vi "Dresden R2R Sputter 03.02.2018 IY24.vi"() -> ()   [LabVIEW 2009] (continued)
        n5019 = case shown="True" w7481 {
          frame #0 {
          }
          frame #1 {
            "ch1_trns_gv_bp2_timer_top" <- TRUE
          }
        }
        n5020 = case shown="True" w7485 {
          frame #0 {
          }
          frame #1 {
            "Gv_timer_top_ch1_2" <- TRUE
          }
        }
        n5021 = case shown="True" w7483 {
          frame #0 {
          }
          frame #1 {
            "ch1_cc_timer_top" <- TRUE
          }
        }
        n5022 = case shown="True" w7482 {
          frame #0 {
          }
          frame #1 {
            "ch1_bg_bv_timer_top" <- TRUE
          }
        }
        n5023 = case shown="True" w7438 {
          frame #0 {
          }
          frame #1 {
            "ch1_sov_Ar_timer_top" <- TRUE
          }
        }
        n5024 = local read "ch1_trns_gv_bp2_timer_top"() -> (w7460:bool)
        n5025 = local read "ch1_bg_bv_timer_top"() -> (w7458:bool)
        n5026 = local read "ch1_sov_Ar_timer_top"() -> (w7440:bool)
        n5027 = local read "Gv_timer_top_ch1_2"() -> (w7461:bool)
        n5028 = Build Array(TRUE, w7484, w7474, w7473, w7472, w7471, w7470, w7451, w7439, w7443, w7417, w7416, w7415) -> (w7524:bool[])
        n5029 = local read "ch1_cc_timer_top"() -> (w7459:bool)
        n5030 = Boolean Array To Number(Boolean array=w7524) -> (number=w7532:u32)
        n5031 = feedback #140() -> (w7468:bool)  [unwired: 1 in]
        n5032 = feedback #141() -> (w7467:bool)  [unwired: 1 in]
        n5033 = feedback #142() -> (w7463:bool)  [unwired: 1 in]
        n5034 = feedback #143() -> (w7441:bool)  [unwired: 1 in]
        n5035 = feedback #144() -> (w7464:bool)  [unwired: 1 in]
        n5036 = Mantissa & Exponent(0:w7532) -> (2:w7528:dbl)  [unwired: 1 out]
        n5037 = case shown="True" w7461 {
          tunnel: [TRUE FALSE] -> w7469
          tunnel: w7468 -> [_ w7585]
          frame #0 {
          }
          frame #1 {
            n5038 = call "Elapsed Time80"("Reset"=w7585) -> ("Elapsed Time (s)"=w7582:dbl)  [unwired: 11 in, 7 out]
            n5039 = Greater?(x=w7582, y=3.0) -> (0:w7583:bool)
            n5040 = In Range and Coerce(upper limit=3.0, x=w7582, lower limit=0.0) -> (In Range?=w7579:bool)  [unwired: 1 out]
            n5041 = Not(x=w7583) -> (.not. x?=w7578:bool)
            n5042 = property on="Gv_timer_top_ch1_2_gui" class="TabCtl (strict)"("Visible"=w7579) -> ()  [unwired: 2 in, 2 out]
            n5043 = local write "Gv_timer_top_ch1_2"(w7578) -> ()
          }
        }
        n5044 = case shown="True" w7460 {
          tunnel: [TRUE FALSE] -> w7466
          tunnel: w7467 -> [_ w7575]
          frame #0 {
          }
          frame #1 {
            n5045 = call "Elapsed Time81"("Reset"=w7575) -> ("Elapsed Time (s)"=w7572:dbl)  [unwired: 11 in, 7 out]
            n5046 = Greater?(x=w7572, y=3.0) -> (0:w7573:bool)
            n5047 = In Range and Coerce(upper limit=3.0, x=w7572, lower limit=0.0) -> (In Range?=w7569:bool)  [unwired: 1 out]
            n5048 = Not(x=w7573) -> (.not. x?=w7568:bool)
            n5049 = local write "ch1_trns_gv_bp2_timer_top"(w7568) -> ()
            n5050 = property on="Ch1_trns_gb_bp2_timer_top_gui" class="TabCtl (strict)"("Visible"=w7569) -> ()  [unwired: 2 in, 2 out]
          }
        }
        n5051 = case shown="True" w7458 {
          tunnel: [TRUE FALSE] -> w7462
          tunnel: w7463 -> [_ w7555]
          frame #0 {
          }
          frame #1 {
            n5052 = call "Elapsed Time83"("Reset"=w7555) -> ("Elapsed Time (s)"=w7552:dbl)  [unwired: 11 in, 7 out]
            n5053 = Greater?(x=w7552, y=3.0) -> (0:w7553:bool)
            n5054 = In Range and Coerce(upper limit=3.0, x=w7552, lower limit=0.0) -> (In Range?=w7548:bool)  [unwired: 1 out]
            n5055 = Not(x=w7553) -> (.not. x?=w7549:bool)
            n5056 = property on="Ch1_bg_bv_timer_top_gui" class="TabCtl (strict)"("Visible"=w7548) -> ()  [unwired: 2 in, 2 out]
            n5057 = local write "ch1_bg_bv_timer_top"(w7549) -> ()
          }
        }
        n5058 = case shown="True" w7440 {
          tunnel: [TRUE FALSE] -> w7442
          tunnel: w7441 -> [_ w7544]
          frame #0 {
          }
          frame #1 {
            n5059 = call "Elapsed Time119"("Reset"=w7544) -> ("Elapsed Time (s)"=w7541:dbl)  [unwired: 11 in, 7 out]
            n5060 = Greater?(x=w7541, y=3.0) -> (0:w7542:bool)
            n5061 = In Range and Coerce(upper limit=3.0, x=w7541, lower limit=0.0) -> (In Range?=w7537:bool)  [unwired: 1 out]
            n5062 = Not(x=w7542) -> (.not. x?=w7538:bool)
            n5063 = property on="Ch1_sov_Ar_timer_top_gui" class="TabCtl (strict)"("Visible"=w7537) -> ()  [unwired: 2 in, 2 out]
            n5064 = local write "ch1_sov_Ar_timer_top"(w7538) -> ()
          }
        }
        n5065 = case shown="True" w7459 {
          tunnel: [TRUE FALSE] -> w7465
          tunnel: w7464 -> [_ w7565]
          frame #0 {
          }
          frame #1 {
            n5066 = call "Elapsed Time82"("Reset"=w7565) -> ("Elapsed Time (s)"=w7562:dbl)  [unwired: 11 in, 7 out]
            n5067 = Greater?(x=w7562, y=3.0) -> (0:w7563:bool)
            n5068 = In Range and Coerce(upper limit=3.0, x=w7562, lower limit=0.0) -> (In Range?=w7559:bool)  [unwired: 1 out]
            n5069 = Not(x=w7563) -> (.not. x?=w7558:bool)
            n5070 = local write "ch1_cc_timer_top"(w7558) -> ()
            n5071 = property on="Ch1_cc_timer_top_gui" class="TabCtl (strict)"("Visible"=w7559) -> ()  [unwired: 2 in, 2 out]
          }
        }
        n5072 = case shown="12" w7528 {
          tunnel: [cluster{"x":i16, "y":i16} {"x"=0, "y"=0} ("origin") cluster{"x":i16, "y":i16} {"x"=75, "y"=463} ("origin") cluster{"x":i16, "y":i16} {"x"=198, "y"=269} ("origin") cluster{"x":i16, "y":i16} {"x"=282, "y"=670} ("origin") cluster{"x":i16, "y":i16} {"x"=420, "y"=648} ("origin") cluster{"x":i16, "y":i16} {"x"=491, "y"=687} ("origin") cluster{"x":i16, "y":i16} {"x"=206, "y"=664} ("origin") cluster{"x":i16, "y":i16} {"x"=383, "y"=718} ("origin") cluster{"x":i16, "y":i16} {"x"=502, "y"=186} ("origin") cluster{"x":i16, "y":i16} {"x"=562, "y"=180} ("origin") cluster{"x":i16, "y":i16} {"x"=250, "y"=166} ("origin") cluster{"x":i16, "y":i16} {"x"=414, "y"=166} ("origin") cluster{"x":i16, "y":i16} {"x"=320, "y"=144} ("origin")] -> w7530
          tunnel: ["" ("text") "GV" ("text") "GV-BP" ("text") "CH-CC" ("text") "BG-BV" ("text") "CH-ATM" ("text") "CH-PG" ("text") "CH-BG" ("text") "SOV-Ar" ("text") "MFC" ("text") "CST-FIX" ("text") "CST-FIX" ("text") "PET-COOL" ("text")] -> w7531
          tunnel: ["" ("DESCRIPTION") "Gate Valve" ("DESCRIPTION") "Gate Valve- By Pass" ("DESCRIPTION") "Chamber-Cold Cathode" ("DESCRIPTION") "Baratron Gauge-Block Valve" ("DESCRIPTION") "Chamber-Atmospheric Switch" ("DESCRIPTION") "Chamber-Pirani Gauge" ("DESCRIPTION") "Chamber-Baratron Gauge" ("DESCRIPTION") "Shut Off Valve-Ar Gas" ("DESCRIPTION") "Mass Flow Control" ("DESCRIPTION") "Casette Fix" ("DESCRIPTION") "Casette Fix" ("DESCRIPTION") "Petfolio Cool " ("DESCRIPTION")] -> w7529
          frame #0 {
          }
          frame #1 {
          }
          frame #2 {
          }
          frame #3 {
          }
          frame #4 {
          }
          frame #5 {
          }
          frame #6 {
          }
          frame #7 {
          }
          frame #8 {
          }
          frame #9 {
          }
          frame #10 {
          }
          frame #11 {
          }
          frame #12 {
          }
        }
        n5073 = local write "DESCRIPTION"(w7529) -> ()
        n5074 = call <vilib>:"Draw Text at Point.vi"("[user-specified font]"=T35 {"Font Name:"="BOLD", "Size"=18, "Strikeout?"=FALSE, "Italic?"=FALSE, "Underline?"=FALSE, "Outline?"=FALSE, "Shadow?"=FALSE, "Bold?"=TRUE} ("[user-specified font] 9"), "desired font(Application)"=T36."User-specified Font", "text"=w7531, "origin"=w7530, "picture"=w7527) -> ("new picture"=w7522:picture)  [unwired: 5 in, 1 out]
      }
    }
    "new picture 7" <- w7254
    n5075 = stacked-sequence {
      tunnel: w7282 -> [w7649 _]
      tunnel: [_ w7738] -> w7269
      tunnel: w7281 -> [w7683 _]
      tunnel: w7280 -> [w7681 _]
      tunnel: w7279 -> [w7676 _]
      tunnel: w7278 -> [w7671 _]
      tunnel: w7277 -> [w7670 _]
      tunnel: w7276 -> [w7661 _]
      tunnel: w7275 -> [w7652 _]
      tunnel: w7274 -> [w7651 _]
      tunnel: w7268 -> [w7635 _]
      tunnel: w7267 -> [w7634 _]
      frame #0 {
        n5076 = Build Array(FALSE ("element"), "chamber1 front piston open drum failed", "chamber1 front piston failed drum open", "chamber1 front piston open") -> (w7687:bool[])
        n5077 = Build Array(FALSE ("element"), "magnetron on ch1") -> (w7666:bool[])
        n5078 = Build Array(FALSE ("element"), "gv front open ch1_2", "gv front failed ch1_2") -> (w7679:bool[])
        n5079 = Build Array(FALSE ("element"), "magnetron water cooled on ch1", "magnetron water cooled failed ch1") -> (w7653:bool[])
        n5080 = Build Array(FALSE ("element"), "Trns_gv_bp2_ch1_fail_front", "Trns_gv_bp2_ch1_on_front") -> (w7640:bool[])
        n5081 = Boolean Array To Number(Boolean array=w7687) -> (number=w7686:u32)
        n5082 = Boolean Array To Number(Boolean array=w7666) -> (number=w7665:u32)
        n5083 = Boolean Array To Number(Boolean array=w7679) -> (number=w7680:u32)
        n5084 = Boolean Array To Number(Boolean array=w7653) -> (number=w7654:u32)
        n5085 = Boolean Array To Number(Boolean array=w7640) -> (number=w7639:u32)
        n5086 = Mantissa & Exponent(0:w7686) -> (2:w7685:dbl)  [unwired: 1 out]
        n5087 = Mantissa & Exponent(0:w7665) -> (2:w7662:dbl)  [unwired: 1 out]
        n5088 = Mantissa & Exponent(0:w7680) -> (2:w7675:dbl)  [unwired: 1 out]
        n5089 = Mantissa & Exponent(0:w7654) -> (2:w7657:dbl)  [unwired: 1 out]
        n5090 = Mantissa & Exponent(0:w7639) -> (2:w7636:dbl)  [unwired: 1 out]
        n5091 = case shown="0, Default" w7685 {
          tunnel: [u32[][] [] ("data (RGB format)") w7700 w7701 w7702] -> w7684
          tunnel: w7683 -> [_ w7700 _ _]
          tunnel: w7681 -> [_ _ w7701 _]
          tunnel: w7671 -> [_ _ _ w7702]
          frame #0 {
          }
          frame #1 {
          }
          frame #2 {
          }
          frame #3 {
          }
        }
        n5092 = case shown="0, Default" w7675 {
          tunnel: [u32[][] [] ("data (RGB format)") w7697 w7698] -> w7677
          tunnel: w7676 -> [_ w7697 _]
          tunnel: w7670 -> [_ _ w7698]
          frame #0 {
          }
          frame #1 {
          }
          frame #2 {
          }
        }
        n5093 = case shown="0, Default" w7662 {
          tunnel: w7661 -> [_ w7695]
          tunnel: [u32[][] [] ("data (RGB format)") w7695] -> w7659
          frame #0 {
          }
          frame #1 {
          }
        }
        n5094 = case shown="0, Default" w7657 {
          tunnel: w7652 -> [_ w7692 _]
          tunnel: [u32[][] [] ("data (RGB format)") w7692 w7693] -> w7658
          tunnel: w7651 -> [_ _ w7693]
          frame #0 {
          }
          frame #1 {
          }
          frame #2 {
          }
        }
        n5095 = case shown="0, Default" w7636 {
          tunnel: w7635 -> [_ w7689 _]
          tunnel: [u32[][] [] ("data (RGB format)") w7689 w7690] -> w7631
          tunnel: w7634 -> [_ _ w7690]
          frame #0 {
          }
          frame #1 {
          }
          frame #2 {
          }
        }
        n5096 = call-poly <vilib>:"Draw Unflattened Pixmap.vi"("top left point(0, 0)"=cluster{"x":i16, "y":i16} {"x"=100, "y"=167}, "data (RGB format)"=w7649) -> ("new picture"=w7647:picture)  [unwired: 7 in]
        n5097 = call-poly <vilib>:"Draw Unflattened Pixmap.vi"("picture"=w7647, "top left point(0, 0)"=cluster{"x":i16, "y":i16} {"x"=187, "y"=296} ("top left point(0, 0) 3"), "data (RGB format)"=w7684) -> ("new picture"=w7678:picture)  [unwired: 6 in]
        n5098 = call-poly <vilib>:"Draw Unflattened Pixmap.vi"("picture"=w7678, "top left point(0, 0)"=cluster{"x":i16, "y":i16} {"x"=98, "y"=311} ("top left point(0, 0) 2"), "data (RGB format)"=w7677) -> ("new picture"=w7660:picture)  [unwired: 6 in]
        n5099 = call-poly <vilib>:"Draw Unflattened Pixmap.vi"("picture"=w7660, "top left point(0, 0)"=cluster{"x":i16, "y":i16} {"x"=296, "y"=587}, "data (RGB format)"=w7659) -> ("new picture"=w7648:picture)  [unwired: 6 in]
        n5100 = call-poly <vilib>:"Draw Unflattened Pixmap.vi"("picture"=w7648, "top left point(0, 0)"=cluster{"x":i16, "y":i16} {"x"=316, "y"=647}, "data (RGB format)"=w7658) -> ("new picture"=w7632:picture)  [unwired: 6 in]
        n5101 = call-poly <vilib>:"Draw Unflattened Pixmap.vi"("picture"=w7632, "top left point(0, 0)"=cluster{"x":i16, "y":i16} {"x"=182, "y"=249}, "data (RGB format)"=w7631) -> ("new picture"=w7633:picture)  [unwired: 6 in]
      }
      frame #1 {
        # "PET COOL"
        # "CST-FIX"
        # "CST-FIX"
        n5102 = property on="new picture 8" class="Pict"() -> ("Mouse"=w7737:T37)  [unwired: 2 in, 2 out]
        n5103 = Unbundle(w7737) -> ("Mouse Position"=w7736:cluster{"X":i32, "Y":i32}, "Mouse Modifiers"=w7735:T38)
        "Mouse Position 8" <- w7736
        n5104 = Unbundle(w7736) -> ("X"=w7704:i32, "Y"=w7703:i32)
        n5105 = Unbundle(w7735) -> ("Button Down"=w7734:bool)  [unwired: 3 out]
        n5106 = In Range and Coerce(upper limit=598, x=w7703, lower limit=319) -> (In Range?=w7764:bool)  [unwired: 1 out]
        n5107 = In Range and Coerce(upper limit=146, x=w7704, lower limit=106) -> (In Range?=w7765:bool)  [unwired: 1 out]
        n5108 = In Range and Coerce(upper limit=275, x=w7703, lower limit=204) -> (In Range?=w7763:bool)  [unwired: 1 out]
        n5109 = In Range and Coerce(upper limit=225, x=w7704, lower limit=192) -> (In Range?=w7762:bool)  [unwired: 1 out]
        n5110 = In Range and Coerce(upper limit=331, x=w7703, lower limit=169) -> (In Range?=w7713:bool)  [unwired: 1 out]
        n5111 = In Range and Coerce(upper limit=382, x=w7704, lower limit=342) -> (In Range?=w7712:bool)  [unwired: 1 out]
        n5112 = In Range and Coerce(upper limit=679, x=w7703, lower limit=639) -> (In Range?=w7752:bool)  [unwired: 1 out]
        n5113 = In Range and Coerce(upper limit=324, x=w7703, lower limit=201) -> (In Range?=w7714:bool)  [unwired: 1 out]
        n5114 = In Range and Coerce(upper limit=425, x=w7704, lower limit=303) -> (In Range?=w7753:bool)  [unwired: 1 out]
        n5115 = In Range and Coerce(upper limit=471, x=w7704, lower limit=446) -> (In Range?=w7715:bool)  [unwired: 1 out]
        n5116 = In Range and Coerce(upper limit=324, x=w7703, lower limit=201) -> (In Range?=w7725:bool)  [unwired: 1 out]
        n5117 = In Range and Coerce(upper limit=275, x=w7704, lower limit=247) -> (In Range?=w7724:bool)  [unwired: 1 out]
        n5118 = And(x=w7765, y=w7764) -> (x .and. y?=w7745:bool)
        n5119 = And(x=w7762, y=w7763) -> (x .and. y?=w7733:bool)
        n5120 = And(x=w7712, y=w7713) -> (x .and. y?=w7705:bool)
        n5121 = And(x=w7753, y=w7752) -> (x .and. y?=w7732:bool)
        n5122 = And(x=w7715, y=w7714) -> (x .and. y?=w7706:bool)
        n5123 = And(x=w7724, y=w7725) -> (x .and. y?=w7707:bool)
        n5124 = And(x=w7734, y=w7745) -> (x .and. y?=w7747:bool)
        n5125 = And(x=w7734, y=w7733) -> (x .and. y?=w7744:bool)
        n5126 = case shown="True" w7747 {
          frame #0 {
          }
          frame #1 {
            "Gv_timer_front_ch1_2" <- TRUE ("Gv_timer_front_ch2_3")
          }
        }
        n5127 = case shown="True" w7744 {
          frame #0 {
          }
          frame #1 {
            "ch1_trns_gv_bp2_timer_front" <- TRUE ("ch2_bv_L_timerl_front")
          }
        }
        n5128 = Build Array(TRUE, w7745, w7733, w7732, w7707, w7706, w7705) -> (w7748:bool[])
        n5129 = local read "ch1_trns_gv_bp2_timer_front"() -> (w7726:bool)
        n5130 = local read "Gv_timer_front_ch1_2"() -> (w7727:bool)
        n5131 = Boolean Array To Number(Boolean array=w7748) -> (number=w7751:u32)
        n5132 = Mantissa & Exponent(0:w7751) -> (2:w7740:dbl)  [unwired: 1 out]
        n5133 = feedback #145() -> (w7728:bool)  [unwired: 1 in]
        n5134 = feedback #146() -> (w7730:bool)  [unwired: 1 in]
        n5135 = case shown="True" w7726 {
          tunnel: [TRUE FALSE] -> w7729
          tunnel: w7728 -> [_ w7778]
          frame #0 {
          }
          frame #1 {
            n5136 = call "Elapsed Time79"("Reset"=w7778) -> ("Elapsed Time (s)"=w7775:dbl)  [unwired: 11 in, 7 out]
            n5137 = Greater?(x=w7775, y=3.0) -> (0:w7776:bool)
            n5138 = In Range and Coerce(upper limit=3.0, x=w7775, lower limit=0.0) -> (In Range?=w7772:bool)  [unwired: 1 out]
            n5139 = Not(x=w7776) -> (.not. x?=w7771:bool)
            n5140 = local write "ch1_trns_gv_bp2_timer_front"(w7771) -> ()
            n5141 = property on="Ch1_trns_gv_bp2_timer_front_gui" class="TabCtl (strict)"("Visible"=w7772) -> ()  [unwired: 2 in, 2 out]
          }
        }
        n5142 = case shown="True" w7727 {
          tunnel: [TRUE FALSE] -> w7731
          tunnel: w7730 -> [_ w7788]
          frame #0 {
          }
          frame #1 {
            n5143 = call "Elapsed Time78"("Reset"=w7788) -> ("Elapsed Time (s)"=w7785:dbl)  [unwired: 11 in, 7 out]
            n5144 = Greater?(x=w7785, y=3.0) -> (0:w7786:bool)
            n5145 = In Range and Coerce(upper limit=3.0, x=w7785, lower limit=0.0) -> (In Range?=w7782:bool)  [unwired: 1 out]
            n5146 = Not(x=w7786) -> (.not. x?=w7781:bool)
            n5147 = local write "Gv_timer_front_ch1_2"(w7781) -> ()
            n5148 = property on="Gv_timer_front_ch1_2_gui" class="TabCtl (strict)"("Visible"=w7782) -> ()  [unwired: 2 in, 2 out]
          }
        }
        n5149 = case shown="6" w7740 {
          tunnel: [cluster{"x":i16, "y":i16} {"x"=0, "y"=0} ("origin") cluster{"x":i16, "y":i16} {"x"=71, "y"=502} ("origin") cluster{"x":i16, "y":i16} {"x"=186, "y"=231} ("origin") cluster{"x":i16, "y":i16} {"x"=353, "y"=707} ("origin") cluster{"x":i16, "y":i16} {"x"=231, "y"=185} ("origin") cluster{"x":i16, "y":i16} {"x"=440, "y"=185} ("origin") cluster{"x":i16, "y":i16} {"x"=327, "y"=149} ("origin")] -> w7742
          tunnel: ["" ("text") "GV" ("text") "GV-BP" ("text") "MG" ("text") "CST-FIX" ("text") "CST-FIX" ("text") "PET-COOL" ("text")] -> w7743
          tunnel: ["" ("DESCRIPTION") "Gate Valve" ("DESCRIPTION") "Gate Valve- By Pass" ("DESCRIPTION") "MAGNETRON" ("DESCRIPTION") "Casette Fix" ("DESCRIPTION") "Casette Fix" ("DESCRIPTION") "Petfolio Cool " ("DESCRIPTION")] -> w7741
          frame #0 {
          }
          frame #1 {
          }
          frame #2 {
          }
          frame #3 {
          }
          frame #4 {
          }
          frame #5 {
          }
          frame #6 {
          }
        }
        n5150 = local write "DESCRIPTION"(w7741) -> ()
        n5151 = call <vilib>:"Draw Text at Point.vi"("[user-specified font]"=T35 {"Font Name:"="BOLD", "Size"=18, "Strikeout?"=FALSE, "Italic?"=FALSE, "Underline?"=FALSE, "Outline?"=FALSE, "Shadow?"=FALSE, "Bold?"=TRUE} ("[user-specified font] 8"), "desired font(Application)"=T36."User-specified Font", "text"=w7743, "origin"=w7742, "picture"=w7739) -> ("new picture"=w7738:picture)  [unwired: 5 in, 1 out]
      }
    }
    "new picture 8" <- w7269
  }
  n5152 = while {
    tunnel: w557 -> [w7853]
    tunnel: w556 -> [w7852]
    tunnel: w555 -> [w7851]
    tunnel: w554 -> [w7850]
    tunnel: w553 -> [w7849]
    tunnel: w552 -> [w7848]
    tunnel: w551 -> [w7847]
    tunnel: w550 -> [w7846]
    tunnel: w549 -> [w7845]
    tunnel: w548 -> [w7844]
    tunnel: w547 -> [w7843]
    tunnel: w546 -> [w7842]
    tunnel: w545 -> [w7841]
    tunnel: w544 -> [w7840]
    tunnel: w225 -> [w7838]
    tunnel: w224 -> [w7837]
    tunnel: w175 -> [w7836]
    tunnel: w174 -> [w7835]
    tunnel: w173 -> [w7834]
    tunnel: w172 -> [w7833]
    tunnel: w171 -> [w7832]
    tunnel: w170 -> [w7831]
    tunnel: w169 -> [w7830]
    tunnel: w168 -> [w7829]
    tunnel: w167 -> [w7828]
    tunnel: w166 -> [w7827]
    tunnel: w165 -> [w7826]
    tunnel: w164 -> [w7825]
    tunnel: w163 -> [w7824]
    tunnel: w162 -> [w7823]
    tunnel: w161 -> [w7822]
    tunnel: w160 -> [w7821]
    tunnel: w126 -> [w7820]
    tunnel: w125 -> [w7819]
    tunnel: w111 -> [w7818]
    tunnel: w110 -> [w7817]
    tunnel: w109 -> [w7816]
    tunnel: w108 -> [w7815]
    stop <- FALSE stop-if-true
    n5153 = stacked-sequence {
      tunnel: w7853 -> [w8340 _]
      tunnel: w7852 -> [w8339 _]
      tunnel: w7851 -> [w8338 _]
      tunnel: w7850 -> [w8337 _]
      tunnel: w7849 -> [w8335 _]
      tunnel: w7848 -> [w8336 _]
      tunnel: w7847 -> [w8334 _]
      tunnel: w7846 -> [w8333 _]
      tunnel: w7845 -> [w8332 _]
      tunnel: [_ w8433] -> w7839
      tunnel: w7838 -> [w8311 _]
      tunnel: w7837 -> [w8310 _]
      tunnel: w7818 -> [w8285 _]
      tunnel: w7817 -> [w8284 _]
      tunnel: w7816 -> [w8283 _]
      tunnel: w7815 -> [w8282 _]
      frame #0 {
        n5154 = Build Array(FALSE ("element"), "ch2_trns_gv_bp2_on_front", "ch2_trns_gv_bp2_fail_front") -> (w8296:bool[])
        n5155 = Build Array(FALSE ("element"), "magnetron on_ch3") -> (w8354:bool[])
        n5156 = Build Array(FALSE ("element"), "chamber2 front piston failed drum open", "chamber2 front piston open drum failed", "chamber2front piston open") -> (w8344:bool[])
        n5157 = Build Array(FALSE ("element"), "gv front open_ch2_3", "gv front failed_ch2_3") -> (w8357:bool[])
        n5158 = Build Array(FALSE ("element"), "ch2_trns_gv_bp_fail_front", "ch2_trns_gv_bp_on_front") -> (w8291:bool[])
        n5159 = Build Array(FALSE ("element"), "magnetron water cooled on_ch2", "magnetron water cooled failed_ch2") -> (w8346:bool[])
        n5160 = Build Array(FALSE ("element"), "gv front failed_ch2_1", "gv front open_ch2_1") -> (w8312:bool[])
        n5161 = Boolean Array To Number(Boolean array=w8296) -> (number=w8297:u32)
        n5162 = Boolean Array To Number(Boolean array=w8354) -> (number=w8353:u32)
        n5163 = Boolean Array To Number(Boolean array=w8344) -> (number=w8343:u32)
        n5164 = Boolean Array To Number(Boolean array=w8357) -> (number=w8358:u32)
        n5165 = Boolean Array To Number(Boolean array=w8291) -> (number=w8302:u32)
        n5166 = Boolean Array To Number(Boolean array=w8346) -> (number=w8347:u32)
        n5167 = Boolean Array To Number(Boolean array=w8312) -> (number=w8313:u32)
        n5168 = Mantissa & Exponent(0:w8297) -> (2:w8298:dbl)  [unwired: 1 out]
        n5169 = Mantissa & Exponent(0:w8302) -> (2:w8301:dbl)  [unwired: 1 out]
        n5170 = Mantissa & Exponent(0:w8353) -> (2:w8352:dbl)  [unwired: 1 out]
        n5171 = Mantissa & Exponent(0:w8343) -> (2:w8342:dbl)  [unwired: 1 out]
        n5172 = Mantissa & Exponent(0:w8358) -> (2:w8355:dbl)  [unwired: 1 out]
        n5173 = Mantissa & Exponent(0:w8313) -> (2:w8314:dbl)  [unwired: 1 out]
        n5174 = Mantissa & Exponent(0:w8347) -> (2:w8348:dbl)  [unwired: 1 out]
        n5175 = case shown="1" w8301 {
          tunnel: [u32[][] [] ("data (RGB format)") w8364 w8365] -> w8300
          tunnel: w8285 -> [_ w8364 _]
          tunnel: w8284 -> [_ _ w8365]
          frame #0 {
          }
          frame #1 {
          }
          frame #2 {
          }
        }
        n5176 = case shown="2" w8298 {
          tunnel: [u32[][] [] ("data (RGB format)") w8361 w8362] -> w8299
          tunnel: w8283 -> [_ w8361 _]
          tunnel: w8282 -> [_ _ w8362]
          frame #0 {
          }
          frame #1 {
          }
          frame #2 {
          }
        }
        n5177 = case shown="1" w8342 {
          tunnel: [u32[][] [] ("data (RGB format)") w8378 w8379 w8380] -> w8341
          tunnel: w8339 -> [_ w8378 _ _]
          tunnel: w8338 -> [_ _ w8379 _]
          tunnel: w8337 -> [_ _ _ w8380]
          frame #0 {
          }
          frame #1 {
          }
          frame #2 {
          }
          frame #3 {
          }
        }
        n5178 = case shown="0, Default" w8314 {
          tunnel: w8311 -> [_ w8367 _]
          tunnel: [u32[][] [] ("data (RGB format)") w8367 w8368] -> w8318
          tunnel: w8310 -> [_ _ w8368]
          frame #0 {
          }
          frame #1 {
          }
          frame #2 {
          }
        }
        n5179 = case shown="1" w8355 {
          tunnel: [u32[][] [] ("data (RGB format)") w8375 w8376] -> w8356
          tunnel: w8336 -> [_ _ w8376]
          tunnel: w8335 -> [_ w8375 _]
          frame #0 {
          }
          frame #1 {
          }
          frame #2 {
          }
        }
        n5180 = case shown="1" w8352 {
          tunnel: [u32[][] [] ("data (RGB format)") w8373] -> w8350
          tunnel: w8334 -> [_ w8373]
          frame #0 {
          }
          frame #1 {
          }
        }
        n5181 = case shown="0, Default" w8348 {
          tunnel: w8333 -> [_ w8370 _]
          tunnel: [u32[][] [] ("data (RGB format)") w8370 w8371] -> w8349
          tunnel: w8332 -> [_ _ w8371]
          frame #0 {
          }
          frame #1 {
          }
          frame #2 {
          }
        }
        n5182 = call-poly <vilib>:"Draw Unflattened Pixmap.vi"("top left point(0, 0)"=cluster{"x":i16, "y":i16} {"x"=93, "y"=169}, "data (RGB format)"=w8340) -> ("new picture"=w8331:picture)  [unwired: 7 in]
        n5183 = call-poly <vilib>:"Draw Unflattened Pixmap.vi"("picture"=w8331, "top left point(0, 0)"=cluster{"x":i16, "y":i16} {"x"=182, "y"=297}, "data (RGB format)"=w8341) -> ("new picture"=w8359:picture)  [unwired: 6 in]
        n5184 = call-poly <vilib>:"Draw Unflattened Pixmap.vi"("picture"=w8359, "top left point(0, 0)"=cluster{"x":i16, "y":i16} {"x"=564, "y"=310}, "data (RGB format)"=w8356) -> ("new picture"=w8351:picture)  [unwired: 6 in]
        n5185 = call-poly <vilib>:"Draw Unflattened Pixmap.vi"("picture"=w8351, "top left point(0, 0)"=cluster{"x":i16, "y":i16} {"x"=282, "y"=593}, "data (RGB format)"=w8350) -> ("new picture"=w8345:picture)  [unwired: 6 in]
        n5186 = call-poly <vilib>:"Draw Unflattened Pixmap.vi"("picture"=w8345, "top left point(0, 0)"=cluster{"x":i16, "y":i16} {"x"=304, "y"=649}, "data (RGB format)"=w8349) -> ("new picture"=w8309:picture)  [unwired: 6 in]
        n5187 = call-poly <vilib>:"Draw Unflattened Pixmap.vi"("picture"=w8309, "top left point(0, 0)"=cluster{"x":i16, "y":i16} {"x"=92, "y"=313}, "data (RGB format)"=w8318) -> ("new picture"=w8286:picture)  [unwired: 6 in]
        n5188 = call-poly <vilib>:"Draw Unflattened Pixmap.vi"("picture"=w8286, "top left point(0, 0)"=cluster{"x":i16, "y":i16} {"x"=175, "y"=251}, "data (RGB format)"=w8300) -> ("new picture"=w8287:picture)  [unwired: 6 in]
        n5189 = call-poly <vilib>:"Draw Unflattened Pixmap.vi"("picture"=w8287, "top left point(0, 0)"=cluster{"x":i16, "y":i16} {"x"=488, "y"=250} ("top left point(0, 0) 2"), "data (RGB format)"=w8299) -> ("new picture"=w8288:picture)  [unwired: 6 in]
      }
      frame #1 {
        # "PET COOL"
        # "CST FIX"
        # "CST FIX"
        n5190 = property on="new picture 5" class="Pict"() -> ("Mouse"=w8468:T37)  [unwired: 2 in, 2 out]
        n5191 = Unbundle(w8468) -> ("Mouse Position"=w8467:cluster{"X":i32, "Y":i32}, "Mouse Modifiers"=w8469:T38)
        "Mouse Position 6" <- w8467
        n5192 = Unbundle(w8469) -> ("Button Down"=w8436:bool)  [unwired: 3 out]
        n5193 = Unbundle(w8467) -> ("X"=w8382:i32, "Y"=w8381:i32)
        n5194 = In Range and Coerce(upper limit=333, x=w8381, lower limit=171) -> (In Range?=w8391:bool)  [unwired: 1 out]
        n5195 = In Range and Coerce(upper limit=382, x=w8382, lower limit=327) -> (In Range?=w8390:bool)  [unwired: 1 out]
        n5196 = In Range and Coerce(upper limit=605, x=w8381, lower limit=324) -> (In Range?=w8460:bool)  [unwired: 1 out]
        n5197 = In Range and Coerce(upper limit=140, x=w8382, lower limit=98) -> (In Range?=w8459:bool)  [unwired: 1 out]
        n5198 = In Range and Coerce(upper limit=600, x=w8381, lower limit=324) -> (In Range?=w8461:bool)  [unwired: 1 out]
        n5199 = In Range and Coerce(upper limit=325, x=w8381, lower limit=203) -> (In Range?=w8392:bool)  [unwired: 1 out]
        n5200 = In Range and Coerce(upper limit=610, x=w8382, lower limit=570) -> (In Range?=w8462:bool)  [unwired: 1 out]
        n5201 = In Range and Coerce(upper limit=474, x=w8382, lower limit=435) -> (In Range?=w8393:bool)  [unwired: 1 out]
        n5202 = In Range and Coerce(upper limit=277, x=w8381, lower limit=252) -> (In Range?=w8450:bool)  [unwired: 1 out]
        n5203 = In Range and Coerce(upper limit=527, x=w8382, lower limit=490) -> (In Range?=w8451:bool)  [unwired: 1 out]
        n5204 = In Range and Coerce(upper limit=325, x=w8381, lower limit=203) -> (In Range?=w8403:bool)  [unwired: 1 out]
        n5205 = In Range and Coerce(upper limit=275, x=w8382, lower limit=235) -> (In Range?=w8402:bool)  [unwired: 1 out]
        n5206 = In Range and Coerce(upper limit=281, x=w8381, lower limit=256) -> (In Range?=w8449:bool)  [unwired: 1 out]
        n5207 = In Range and Coerce(upper limit=210, x=w8382, lower limit=185) -> (In Range?=w8448:bool)  [unwired: 1 out]
        n5208 = In Range and Coerce(upper limit=685, x=w8381, lower limit=641) -> (In Range?=w8438:bool)  [unwired: 1 out]
        n5209 = In Range and Coerce(upper limit=418, x=w8382, lower limit=283) -> (In Range?=w8439:bool)  [unwired: 1 out]
        n5210 = And(x=w8390, y=w8391) -> (x .and. y?=w8383:bool)
        n5211 = And(x=w8459, y=w8460) -> (x .and. y?=w8423:bool)
        n5212 = And(x=w8462, y=w8461) -> (x .and. y?=w8427:bool)
        n5213 = And(x=w8393, y=w8392) -> (x .and. y?=w8384:bool)
        n5214 = And(x=w8451, y=w8450) -> (x .and. y?=w8422:bool)
        n5215 = And(x=w8402, y=w8403) -> (x .and. y?=w8385:bool)
        n5216 = And(x=w8448, y=w8449) -> (x .and. y?=w8421:bool)
        n5217 = And(x=w8439, y=w8438) -> (x .and. y?=w8420:bool)
        n5218 = And(x=w8436, y=w8427) -> (x .and. y?=w8429:bool)
        n5219 = And(x=w8436, y=w8423) -> (x .and. y?=w8426:bool)
        n5220 = And(x=w8436, y=w8422) -> (x .and. y?=w8425:bool)
        n5221 = And(x=w8436, y=w8421) -> (x .and. y?=w8424:bool)
        n5222 = case shown="True" w8429 {
          frame #0 {
          }
          frame #1 {
            "Gv_timer_front_ch2_1" <- TRUE ("Gv_timer_front_ch2_3")
          }
        }
        n5223 = case shown="True" w8426 {
          frame #0 {
          }
          frame #1 {
            "Gv_timer_front_ch2_3" <- TRUE ("Gv_timer_front_ch2_1")
          }
        }
        n5224 = case shown="True" w8425 {
          frame #0 {
          }
          frame #1 {
            "ch2_trns_gv_bp_timer_front" <- TRUE ("ch2_bv_R_timer_front")
          }
        }
        n5225 = case shown="True" w8424 {
          frame #0 {
          }
          frame #1 {
            "ch2_trns_gv_bp2_timer_front" <- TRUE ("ch2_bv_L_timerl_front")
          }
        }
        n5226 = Build Array(TRUE, w8427, w8423, w8422, w8421, w8420, w8385, w8384, w8383) -> (w8430:bool[])
        n5227 = local read "ch2_trns_gv_bp_timer_front"() -> (w8405:bool)
        n5228 = local read "Gv_timer_front_ch2_3"() -> (w8406:bool)
        n5229 = local read "ch2_trns_gv_bp2_timer_front"() -> (w8404:bool)
        n5230 = local read "Gv_timer_front_ch2_1"() -> (w8407:bool)
        n5231 = Boolean Array To Number(Boolean array=w8430) -> (number=w8435:u32)
        n5232 = Mantissa & Exponent(0:w8435) -> (2:w8416:dbl)  [unwired: 1 out]
        n5233 = feedback #147() -> (w8414:bool)  [unwired: 1 in]
        n5234 = feedback #148() -> (w8413:bool)  [unwired: 1 in]
        n5235 = feedback #149() -> (w8410:bool)  [unwired: 1 in]
        n5236 = feedback #150() -> (w8409:bool)  [unwired: 1 in]
        n5237 = case shown="True" w8407 {
          tunnel: [TRUE FALSE] -> w8415
          tunnel: w8414 -> [_ w8508]
          frame #0 {
          }
          frame #1 {
            n5238 = call "Elapsed Time67"("Reset"=w8508) -> ("Elapsed Time (s)"=w8505:dbl)  [unwired: 11 in, 7 out]
            n5239 = Greater?(x=w8505, y=3.0) -> (0:w8506:bool)
            n5240 = In Range and Coerce(upper limit=3.0, x=w8505, lower limit=0.0) -> (In Range?=w8501:bool)  [unwired: 1 out]
            n5241 = Not(x=w8506) -> (.not. x?=w8502:bool)
            n5242 = local write "Gv_timer_front_ch2_1"(w8502) -> ()
            n5243 = property on="Gv_timer_front_ch2_1_gui" class="TabCtl (strict)"("Visible"=w8501) -> ()  [unwired: 2 in, 2 out]
          }
        }
        n5244 = case shown="True" w8406 {
          tunnel: [TRUE FALSE] -> w8412
          tunnel: w8413 -> [_ w8498]
          frame #0 {
          }
          frame #1 {
            n5245 = call "Elapsed Time68"("Reset"=w8498) -> ("Elapsed Time (s)"=w8495:dbl)  [unwired: 11 in, 7 out]
            n5246 = Greater?(x=w8495, y=3.0) -> (0:w8496:bool)
            n5247 = In Range and Coerce(upper limit=3.0, x=w8495, lower limit=0.0) -> (In Range?=w8491:bool)  [unwired: 1 out]
            n5248 = Not(x=w8496) -> (.not. x?=w8492:bool)
            n5249 = local write "Gv_timer_front_ch2_3"(w8492) -> ()
            n5250 = property on="Gv_timer_front_ch2_3_gui" class="TabCtl (strict)"("Visible"=w8491) -> ()  [unwired: 2 in, 2 out]
          }
        }
        n5251 = case shown="True" w8405 {
          tunnel: [TRUE FALSE] -> w8411
          tunnel: w8410 -> [_ w8488]
          frame #0 {
          }
          frame #1 {
            n5252 = call "Elapsed Time69"("Reset"=w8488) -> ("Elapsed Time (s)"=w8485:dbl)  [unwired: 11 in, 7 out]
            n5253 = Greater?(x=w8485, y=3.0) -> (0:w8486:bool)
            n5254 = In Range and Coerce(upper limit=3.0, x=w8485, lower limit=0.0) -> (In Range?=w8481:bool)  [unwired: 1 out]
            n5255 = Not(x=w8486) -> (.not. x?=w8482:bool)
            n5256 = local write "ch2_trns_gv_bp_timer_front"(w8482) -> ()
            n5257 = property on="Ch2_trns_gv_bp_timer_front_gui" class="TabCtl (strict)"("Visible"=w8481) -> ()  [unwired: 2 in, 2 out]
          }
        }
        n5258 = case shown="True" w8404 {
          tunnel: [TRUE FALSE] -> w8408
          tunnel: w8409 -> [_ w8478]
          frame #0 {
          }
          frame #1 {
            n5259 = call "Elapsed Time70"("Reset"=w8478) -> ("Elapsed Time (s)"=w8475:dbl)  [unwired: 11 in, 7 out]
            n5260 = Greater?(x=w8475, y=3.0) -> (0:w8476:bool)
            n5261 = In Range and Coerce(upper limit=3.0, x=w8475, lower limit=0.0) -> (In Range?=w8471:bool)  [unwired: 1 out]
            n5262 = Not(x=w8476) -> (.not. x?=w8472:bool)
            n5263 = local write "ch2_trns_gv_bp2_timer_front"(w8472) -> ()
            n5264 = property on="Ch2_trns_gv_bp2_front_gui" class="TabCtl (strict)"("Visible"=w8471) -> ()  [unwired: 2 in, 2 out]
          }
        }
        n5265 = case shown="6" w8416 {
          tunnel: [cluster{"x":i16, "y":i16} {"x"=0, "y"=0} ("origin") cluster{"x":i16, "y":i16} {"x"=629, "y"=455} ("origin") cluster{"x":i16, "y":i16} {"x"=52, "y"=455} ("origin") cluster{"x":i16, "y":i16} {"x"=494, "y"=235} ("origin") cluster{"x":i16, "y":i16} {"x"=176, "y"=238} ("origin") cluster{"x":i16, "y":i16} {"x"=342, "y"=709} ("origin") cluster{"x":i16, "y":i16} {"x"=233, "y"=182} ("origin") cluster{"x":i16, "y":i16} {"x"=323, "y"=152} ("origin") cluster{"x":i16, "y":i16} {"x"=485, "y"=182} ("origin")] -> w8418
          tunnel: ["" ("text") "GV" ("text") "GV" ("text") "GV-BP" ("text") "GV-BP" ("text") "MG" ("text") "CST-FIX" ("text") "PET-COOL" ("text") "CST-FIX" ("text")] -> w8419
          tunnel: ["" ("DESCRIPTION") "Gate Valve" ("DESCRIPTION") "Gate Valve" ("DESCRIPTION") "Gate Valve- By Pass" ("DESCRIPTION") "Gate Valve- By Pass" ("DESCRIPTION") "MAGNETRON" ("DESCRIPTION") "Casette Fix" ("DESCRIPTION") "Petfolio Cool" ("DESCRIPTION") "Casette Fix" ("DESCRIPTION")] -> w8417
          frame #0 {
          }
          frame #1 {
          }
          frame #2 {
          }
          frame #3 {
          }
          frame #4 {
          }
          frame #5 {
          }
          frame #6 {
          }
          frame #7 {
          }
          frame #8 {
          }
        }
        n5266 = local write "DESCRIPTION"(w8417) -> ()
        n5267 = call <vilib>:"Draw Text at Point.vi"("[user-specified font]"=T35 {"Font Name:"="BOLD", "Size"=18, "Strikeout?"=FALSE, "Italic?"=FALSE, "Underline?"=FALSE, "Outline?"=FALSE, "Shadow?"=FALSE, "Bold?"=TRUE} ("[user-specified font] 6"), "desired font(Application)"=T36."User-specified Font", "text"=w8419, "origin"=w8418, "picture"=w8434) -> ("new picture"=w8433:picture)  [unwired: 5 in, 1 out]
      }
    }
    "new picture 5" <- w7839
    n5268 = stacked-sequence {
      tunnel: w7844 -> [w7969 _]
      tunnel: w7843 -> [w7968 _]
      tunnel: w7842 -> [w7967 _]
      tunnel: w7841 -> [w7966 _]
      tunnel: w7840 -> [w7965 _]
      tunnel: w7836 -> [w7892 _]
      tunnel: w7835 -> [w7891 _]
      tunnel: w7834 -> [w7890 _]
      tunnel: w7833 -> [w7889 _]
      tunnel: w7832 -> [w7888 _]
      tunnel: w7831 -> [w7887 _]
      tunnel: w7830 -> [w7886 _]
      tunnel: w7829 -> [w7885 _]
      tunnel: w7828 -> [w7884 _]
      tunnel: w7827 -> [w7883 _]
      tunnel: w7826 -> [w7882 _]
      tunnel: w7825 -> [w7881 _]
      tunnel: w7824 -> [w7880 _]
      tunnel: w7823 -> [w7879 _]
      tunnel: w7822 -> [w7878 _]
      tunnel: w7821 -> [w7877 _]
      tunnel: w7820 -> [w7859 _]
      tunnel: w7819 -> [w7858 _]
      tunnel: [_ w8071] -> w7814
      frame #0 {
        n5269 = Build Array(FALSE ("element"), "chamber 2top piston failed", "chamber 2top piston open") -> (w7973:bool[])
        n5270 = Build Array(FALSE ("element"), "gv top failed_ch2_1", "gv top_open_ch2_1") -> (w7900:bool[])
        n5271 = Build Array(FALSE ("element"), "ch2_atm_fail_top", "ch2_atm_on_top") -> (w7952:bool[])
        n5272 = Build Array(FALSE ("element"), "ch2_pg_fail_top", "ch2_pg_on_top") -> (w7945:bool[])
        n5273 = Build Array(FALSE ("element"), "ch2_cc_fail_top", "ch2_cc_on_top") -> (w7937:bool[])
        n5274 = Build Array(FALSE ("element"), "ch2_bg_fail_top", "ch2_bg_on_top") -> (w7929:bool[])
        n5275 = Build Array(FALSE ("element"), "gv top on_ch2_3", "gv top failed_ch2_3") -> (w7974:bool[])
        n5276 = Build Array(FALSE ("element"), "ch2_bg_bv_fail_top", "ch2_bg_bv_on_top") -> (w7921:bool[])
        n5277 = Build Array(FALSE ("element"), "ch2_sov_Ar_on_top", "ch2_sov_Ar_fail_top") -> (w7905:bool[])
        n5278 = Build Array(FALSE ("element"), "Ch2_trns_gv_bp_on_top", "Ch2_trns_gv_bp_fail_top") -> (w7913:bool[])
        n5279 = Build Array(FALSE ("element"), "Ch2_trns_gv_bp2_top", "Ch2_trns_gv_bp2_fail_top") -> (w7863:bool[])
        n5280 = Boolean Array To Number(Boolean array=w7973) -> (number=w7972:u32)
        n5281 = Boolean Array To Number(Boolean array=w7900) -> (number=w7899:u32)
        n5282 = Boolean Array To Number(Boolean array=w7952) -> (number=w7951:u32)
        n5283 = Boolean Array To Number(Boolean array=w7945) -> (number=w7946:u32)
        n5284 = Boolean Array To Number(Boolean array=w7937) -> (number=w7936:u32)
        n5285 = Boolean Array To Number(Boolean array=w7929) -> (number=w7928:u32)
        n5286 = Boolean Array To Number(Boolean array=w7974) -> (number=w7975:u32)
        n5287 = Boolean Array To Number(Boolean array=w7921) -> (number=w7922:u32)
        n5288 = Boolean Array To Number(Boolean array=w7905) -> (number=w7906:u32)
        n5289 = Boolean Array To Number(Boolean array=w7913) -> (number=w7912:u32)
        n5290 = Boolean Array To Number(Boolean array=w7863) -> (number=w7864:u32)
        n5291 = Mantissa & Exponent(0:w7972) -> (2:w7971:dbl)  [unwired: 1 out]
        n5292 = Mantissa & Exponent(0:w7899) -> (2:w7898:dbl)  [unwired: 1 out]
        n5293 = Mantissa & Exponent(0:w7951) -> (2:w7950:dbl)  [unwired: 1 out]
        n5294 = Mantissa & Exponent(0:w7946) -> (2:w7947:dbl)  [unwired: 1 out]
        n5295 = Mantissa & Exponent(0:w7936) -> (2:w7935:dbl)  [unwired: 1 out]
        n5296 = Mantissa & Exponent(0:w7928) -> (2:w7927:dbl)  [unwired: 1 out]
        n5297 = Mantissa & Exponent(0:w7975) -> (2:w7976:dbl)  [unwired: 1 out]
        n5298 = Mantissa & Exponent(0:w7922) -> (2:w7923:dbl)  [unwired: 1 out]
        n5299 = Mantissa & Exponent(0:w7906) -> (2:w7907:dbl)  [unwired: 1 out]
        n5300 = Mantissa & Exponent(0:w7912) -> (2:w7911:dbl)  [unwired: 1 out]
        n5301 = Mantissa & Exponent(0:w7864) -> (2:w7865:dbl)  [unwired: 1 out]
        n5302 = case shown="1" w7971 {
          tunnel: [u32[][] [] ("data (RGB format)") w8012 w8014] -> w7970
          tunnel: w7968 -> [_ w8012 _]
          tunnel: w7967 -> [_ _ w8014]
          tunnel: [cluster{"x":i16, "y":i16} {"x"=0, "y"=0} ("top left point(0, 0) 3") cluster{"x":i16, "y":i16} {"x"=100, "y"=167} ("top left point(0, 0) 3") cluster{"x":i16, "y":i16} {"x"=100, "y"=168} ("top left point(0, 0) 3")] -> w7957
          frame #0 {
          }
          frame #1 {
          }
          frame #2 {
          }
        }
        n5303 = case shown="0, Default" w7898 {
          tunnel: [u32[][] [] ("data (RGB format)") w8004 w8005] -> w7897
          tunnel: w7892 -> [_ w8004 _]
          tunnel: w7891 -> [_ _ w8005]
          frame #0 {
          }
          frame #1 {
          }
          frame #2 {
          }
        }
        n5304 = case shown="2" w7976 {
          tunnel: [u32[][] [] ("data (RGB format)") w8007 w8008] -> w7977
          tunnel: w7966 -> [_ w8007 _]
          tunnel: w7965 -> [_ _ w8008]
          frame #0 {
          }
          frame #1 {
          }
          frame #2 {
          }
        }
        n5305 = case shown="2" w7950 {
          tunnel: w7890 -> [_ w8001 _]
          tunnel: [u32[][] [] ("data (RGB format)") w8001 w8002] -> w7949
          tunnel: w7889 -> [_ _ w8002]
          frame #0 {
          }
          frame #1 {
          }
          frame #2 {
          }
        }
        n5306 = case shown="0, Default" w7947 {
          tunnel: w7888 -> [_ w7998 _]
          tunnel: [u32[][] [] ("data (RGB format)") w7998 w7999] -> w7948
          tunnel: w7887 -> [_ _ w7999]
          frame #0 {
          }
          frame #1 {
          }
          frame #2 {
          }
        }
        n5307 = case shown="1" w7935 {
          tunnel: w7886 -> [_ w7995 _]
          tunnel: [u32[][] [] ("data (RGB format)") w7995 w7996] -> w7934
          tunnel: w7885 -> [_ _ w7996]
          frame #0 {
          }
          frame #1 {
          }
          frame #2 {
          }
        }
        n5308 = case shown="0, Default" w7927 {
          tunnel: w7884 -> [_ w7992 _]
          tunnel: [u32[][] [] ("data (RGB format)") w7992 w7993] -> w7926
          tunnel: w7883 -> [_ _ w7993]
          frame #0 {
          }
          frame #1 {
          }
          frame #2 {
          }
        }
        n5309 = case shown="2" w7923 {
          tunnel: [u32[][] [] ("data (RGB format)") w7989 w7990] -> w7924
          tunnel: w7881 -> [_ _ w7990]
          tunnel: w7882 -> [_ w7989 _]
          frame #0 {
            (unwired) cluster{"x":i16, "y":i16} {"x"=0, "y"=0} ("top left point(0, 0) 2")
          }
          frame #1 {
          }
          frame #2 {
          }
        }
        n5310 = case shown="0, Default" w7907 {
          tunnel: w7878 -> [_ w7983 _]
          tunnel: [u32[][] [] ("data (RGB format)") w7983 w7984] -> w7908
          tunnel: w7877 -> [_ _ w7984]
          frame #0 {
          }
          frame #1 {
          }
          frame #2 {
          }
        }
        n5311 = case shown="0, Default" w7911 {
          tunnel: w7880 -> [_ w7986 _]
          tunnel: [u32[][] [] ("data (RGB format)") w7986 w7987] -> w7910
          tunnel: w7879 -> [_ _ w7987]
          frame #0 {
          }
          frame #1 {
          }
          frame #2 {
          }
        }
        n5312 = case shown="0, Default" w7865 {
          tunnel: w7859 -> [_ w7980 _]
          tunnel: [u32[][] [] ("data (RGB format)") w7980 w7981] -> w7866
          tunnel: w7858 -> [_ _ w7981]
          frame #0 {
          }
          frame #1 {
          }
          frame #2 {
          }
        }
        n5313 = call-poly <vilib>:"Draw Unflattened Pixmap.vi"("top left point(0, 0)"=cluster{"x":i16, "y":i16} {"x"=100, "y"=167}, "data (RGB format)"=w7969) -> ("new picture"=w7958:picture)  [unwired: 7 in]
        n5314 = call-poly <vilib>:"Draw Unflattened Pixmap.vi"("picture"=w7958, "top left point(0, 0)"=w7957, "data (RGB format)"=w7970) -> ("new picture"=w7978:picture)  [unwired: 6 in]
        n5315 = call-poly <vilib>:"Draw Unflattened Pixmap.vi"("picture"=w7978, "top left point(0, 0)"=cluster{"x":i16, "y":i16} {"x"=571, "y"=342} ("top left point(0, 0) 3"), "data (RGB format)"=w7977) -> ("new picture"=w7893:picture)  [unwired: 6 in]
        n5316 = call-poly <vilib>:"Draw Unflattened Pixmap.vi"("picture"=w7893, "top left point(0, 0)"=cluster{"x":i16, "y":i16} {"x"=100, "y"=342} ("top left point(0, 0) 2"), "data (RGB format)"=w7897) -> ("new picture"=w7956:picture)  [unwired: 6 in]